vi "01 Dryer_Performance_SM.vi"() -> ()   [LabVIEW 2012] (continued)
        n146 = Concatenate Strings(w279, w280, w267, w263) -> (w272:string)
        n147 = Build Array (concatenate)(w278, w281, w262) -> (w260:string[])
        n148 = String Length(string=w272) -> (length=w277:i32)
        n149 = Decrement(x=w277) -> (x-1=w271:i32)
        n150 = String Subset(string=w272, offset (0)=w271, length (rest)=1 ("length (rest)")) -> (substring=w275:string)
        n151 = Equal?(x=w275, y=",") -> (x = y?=w273:bool)
        n152 = case shown="True" w273 {
          tunnel: w272 -> [w321 w325]
          tunnel: w271 -> [_ w323]
          tunnel: [w321 w322] -> w261
          frame False {
          }
          frame True {
            n153 = String Subset(string=w325, offset (0)=0, length (rest)=w323) -> (substring=w322:string)
          }
        }
        n154 = call "Agilent Sort Channels.vi"("Agilent Chanel List"=w261, "Agilent Label List"=w260) -> ("Sorted Channels"=w259:string, "Sorted Labels Array"=w256:string[])  [unwired: 12 in]
        n155 = local write "DAQ Chanel List"(w259) -> ()
        n156 = Bundle By Name(cluster=w283, "DAQ Chan List"=w259, "DAQ Label List"=w256) -> (w282:T22)
        n157 = call <vilib>:"Add State(s) to Queue__jki_lib_state_machine.vi"("State(s) in (\"\")"=w286) -> ("States Out"=w285:string)  [unwired: 14 in]
        n158 = local write "DAQ Label List"(w256) -> ()
      }
      frame "Initialize CDAQ Channels" {
        # "if ends in , remove it"
        n159 = global read "Global Test Variables DPT.vi" "Globals for Dryer Performance Test"() -> (w336:T9)
        n160 = local read "cDAQ"() -> (w327:bool)
        n161 = Unbundle By Name(w336) -> ("cDAQ Array Locations.Scale Channel"=w335:string, "cDAQ Array Locations.RH Chan"=w334:string, "cDAQ Array Locations.Temp Chan"=w333:string, "Test Setup.Gas Enabled"=w328:bool, "cDAQ Array Locations.Gas Pressure"=w332:string, "cDAQ Array Locations.Gas Temperature"=w331:string, "cDAQ Array Locations.Barometric Pressure"=w330:string, "cDAQ Array Locations.Gas Feedback Chan"=w329:string)
        n162 = call "Panel DPT Channel Test Labels.vi"("CDAQ?"=w327) -> ("Chanel List"=w340:string, "Label Array"=w358:string[])  [unwired: 12 in, 1 out]
        n163 = local write "TC Chanel List"(w340) -> ()
        n164 = local read "USB Weight?"() -> (w345:bool)
        n165 = Search and Replace String(replace all?=TRUE ("replace all? (F)"), input string=w340, search string=",") -> (number of replacements=w347:i32)  [unwired: 5 in, 3 out]
        n166 = call "Panel DPT Voltage Labels.vi"("Chanel List In"=w340, "CDAQ?"=w327, "Label List In"=w358) -> ("Chanel List Out"=w359:string, "Label List Out"=w357:string[], "Stream DC to File(out)?"=→"Stream DC to File?":bool)  [unwired: 10 in]
        n167 = Increment(x=w347) -> (x+1=w339:i32)
        n168 = case shown="False" w345 {
          tunnel: [string[] ["Weight", "Chamber RH", "Chamber Temp"] ("Label List 2") string[] ["cDAQ Weight", "Chamber RH", "Chamber Temp"] ("Label List 2")] -> w365
          tunnel: [w384 w389] -> w346
          tunnel: w335 -> [w382 w388]
          tunnel: w334 -> [w381 w387]
          tunnel: w333 -> [w380 w386]
          frame False {
            w383 = "," ("string")
            n169 = Concatenate Strings(w382, w383, w381, w383, w380) -> (w384:string)
          }
          frame True {
            w390 = "," ("string")
            n170 = Concatenate Strings(w388, w390, w387, w390, w386) -> (w389:string)
          }
        }
        n171 = local write "Number of TCs"(w339) -> ()
        n172 = String Length(string=w359) -> (length=w364:i32)
        n173 = Greater Than 0?(x=w364) -> (x > 0?=w361:bool)
        n174 = Select(t=",", s=w361, f="") -> (s? t:f=w360:string)
        n175 = case shown="True" w328 {
          tunnel: ["" w379] -> w344
          tunnel: [string[] [] ("Label List 2") string[] ["Gas Pressure", "Gas Temperature", "Barometric Pressure", "Gas Feedback"] ("Label List 2")] -> w343
          tunnel: w332 -> [_ w376]
          tunnel: w331 -> [_ w375]
          tunnel: w330 -> [_ w374]
          tunnel: w329 -> [_ w373]
          frame False {
          }
          frame True {
            w377 = "," ("string")
            n176 = Concatenate Strings(w377, w376, w377, w375, w377, w374, w377, w373) -> (w379:string)
          }
        }
        n177 = Concatenate Strings(w359, w360, w346, w344) -> (w351:string)
        n178 = Build Array (concatenate)(w357, w365, w343) -> (w341:string[])
        n179 = String Length(string=w351) -> (length=w356:i32)
        n180 = Decrement(x=w356) -> (x-1=w350:i32)
        n181 = String Subset(string=w351, offset (0)=w350, length (rest)=1 ("length (rest)")) -> (substring=w354:string)
        n182 = Equal?(x=w354, y=",") -> (x = y?=w352:bool)
        n183 = case shown="True" w352 {
          tunnel: w351 -> [w392 w396]
          tunnel: w350 -> [_ w394]
          tunnel: [w392 w393] -> w342
          frame False {
          }
          frame True {
            n184 = String Subset(string=w396, offset (0)=0, length (rest)=w394) -> (substring=w393:string)
          }
        }
        n185 = call "Agilent Sort Channels.vi"("Agilent Chanel List"=w342, "Agilent Label List"=w341) -> ("Sorted Channels"=w338:string, "Sorted Labels Array"=w337:string[])  [unwired: 12 in]
        n186 = Bundle By Name(cluster=w367, "DAQ Chan List"=w338, "DAQ Label List"=w337) -> (w366:T22)
        n187 = call <vilib>:"Add State(s) to Queue__jki_lib_state_machine.vi"("State(s) in (\"\")"=w370) -> ("States Out"=w369:string)  [unwired: 14 in]
        n188 = local write "DAQ Chanel List"(w338) -> ()
        n189 = local write "DAQ Label List"(w337) -> ()
      }
      frame "----Iniialize Equip-----" {
        # "Do not put any code in this frame.\n(It is a separator no-op. You can make a copy of this frame to create a new Data frame)"
        n190 = call <vilib>:"Add State(s) to Queue__jki_lib_state_machine.vi"("State(s) in (\"\")"=w400) -> ("States Out"=w399:string)  [unwired: 14 in]
      }
      frame "Initialize Equipment" {
        w405 = 4  # Invalid IP Address Length Size
        # "Panel to enter drum volume, MA filter, and scale temp coeff.  \nDrum volume needs to be experimentally determined, depending on a heated run with no clothes.\nThis data is processed with anther program.\n(FIXME, maybe automatically generate this?)"
        n191 = global read "Global Test Variables DPT.vi" "Globals for Dryer Performance Test"() -> (w417:T9)
        n192 = Unbundle By Name(w417) -> ("Test Setup.CompVolume"=w402:dbl, "Test Setup.CDAQ"=w413:bool, "Test Setup.34970"=w412:bool, "Test Setup.34980"=w411:bool, "Test Setup.MA Filter Size"=w408:i32, "Test Setup.RH-IP"=w407:string)
        n193 = Unbundle By Name(w428) -> ("Equipment"=w429:T6)
        n194 = String Length(string=w407) -> (length=w406:i32)
        n195 = Greater?(x=w406, y=w405) -> (0:→"ITHX RH Sensor":bool)
        n196 = local read "Use Smoothing"() -> (w418:bool)
        n197 = local write "MA Filter Size"(w408) -> ()
        n198 = Build Array(w413, w412, w411) -> (w410:bool[])
        n199 = Boolean Array To Number(Boolean array=w410) -> (number=w409:u32)
        n200 = case shown="1" w409 {
          tunnel: [" Init: Power Analyzer\nInit: Power\nInit: Gas\nInit: 34970" ("State(s) in Front (\"\")") " Init: Power Analyzer\nInit: Power\nInit: Gas\nInit: CDAQ" ("State(s) in Front (\"\")") " Init: Power Analyzer\nInit: Power\nInit: Gas\nInit: Agilent" ("State(s) in Front (\"\")")] -> w416
          tunnel: [refnum<visa-resource-name> "AGILENT-34970A" ("VISA resource name") refnum<visa-resource-name> "AGILENT-34970" ("VISA resource name") refnum<visa-resource-name> "AGILENT-34980A" ("VISA resource name")] -> w415
          tunnel: [refnum<visa-resource-name> "WT230" ("Com Power") refnum<visa-resource-name> "WT500" ("Com Power") refnum<visa-resource-name> "WT500" ("Com Power")] -> w414
          frame 2, Default {
          }
          frame 1 {
          }
          frame 4 {
          }
        }
        n201 = Bundle By Name(cluster=w429, "Com Agilent"=w415, "Com Flow Computer"=refnum<visa-resource-name> "COM1", "Com Power Meter"=w414, "Com Power Supply"=refnum<visa-resource-name> "CHROMA") -> (w426:T6)
        "Equipment" <- w426
        n202 = disable-structure shown="Enabled" {
          disable-tunnel: w423 -> [w438 _]
          disable-tunnel: [w437 _] -> w422
          disable-tunnel: [w436 0.0 ("Scale Temp Coeff")] -> w421
          disable-tunnel: [w435 13.0 ("Drum Volume")] -> w401
          disable-tunnel: [w434 w439] -> w419
          disable-tunnel: string[][] [["MA Filter Size", "40"], ["Scale Temp Coeff", "0"], ["Drum Volume", "13"]] ("appended array") -> [_ w439]
          disable-tunnel: w402 -> [w433 _]
          frame Enabled {
            n203 = call "Panel Averaging Values.vi"("Default volume value"=w433, "Error In"=w438) -> ("Scale Temp Coeff Out"=w436:dbl, "Drum Volume"=w435:dbl, "Out Strings"=w434:string[][], "Error Out"=w437:errorcluster)  [unwired: 9 in, 1 out]
          }
          frame Disabled {
          }
        }
        n204 = case shown="True" w418 {
          tunnel: [w451 w455] -> w420
          tunnel: w419 -> [w451 w454]
          frame False {
          }
          frame True {
            n205 = Insert Into Array(array=w454, index (row)=0, new element=string[] ["Smoothing Used"] ("new element/subarray")) -> (w455:string[][])  [unwired: 1 in]
          }
        }
        n206 = Bundle By Name(cluster=w428, "Equipment"=w426, "Start Header Data"=w420) -> (w427:T22)
        n207 = local write "Scale Temp Coeff"(w421) -> ()
        n208 = local write "Drum Volume"(w401) -> ()
        n209 = case shown="No Error" w422 {
          selector: w422 -> [_ w457]
          tunnel: [w456 "Macro: Exit" ("State(s) in Front (\"\")")] -> w430
          tunnel: w416 -> [w456 _]
          frame No Error {
          }
          frame Error {
            n210 = call <vilib>:"Simple Error Handler.vi"("error in (no error)"=w457) -> ()  [unwired: 4 in, 5 out]
          }
        }
        n211 = call <vilib>:"Add State(s) to Queue__jki_lib_state_machine.vi"("State(s) in Front (\"\")"=w430, "State(s) in (\"\")"=w432) -> ("States Out"=w431:string)  [unwired: 13 in]
      }
      frame "Init: Power" {
        # "Sets the Chroma power supply output, and reads the voltages with the WT500 to make sure that the \nPower is in range.\n\nOutputs dryer type to globals.  Tests the voltage settings.  Sets the Supply Voltage output variable."
        n212 = local read "Simulate"() -> (w468:bool)
        n213 = Unbundle By Name(w461) -> ("Equipment.Com Power Meter"=w463:refnum<visa-resource-name>, "Equipment.Com Power Supply"=w470:refnum<visa-resource-name>)
        n214 = global read "Global Test Variables DPT.vi" "Globals for Dryer Performance Test"() -> (w462:T9)
        n215 = case shown="False" w468 {
          tunnel: w470 -> [w495 _]
          tunnel: [w491 w541] -> w466
          tunnel: [w484 "120" ("Supply Voltage:")] -> w469
          tunnel: w467 -> [w494 w541]
          tunnel: w463 -> [w493 _]
          tunnel: w462 -> [w487 _]
          tunnel: [w484 "Electric" ("Chroma Power Setting Out")] -> w459
          frame False {
            n216 = call "Panel Power Setting.vi"() -> ("Dryer Type Out"=w485:string, "Chroma Power Setting Out"=w484:string)  [unwired: 14 in]
            n217 = case shown="\"120\", Default" w484 {
              tunnel: [w506 _ w509 w511] -> w479
              tunnel: [TRUE FALSE TRUE TRUE] -> w478
              frame "120", Default {
                w506 = T19[] [enum."Initialize", enum."Output On 120"] items=["Initialize", "Output On 120", "Output On 240", "Output On 208", "Output Off", "Status", "Send Command", "Track Current"]
              }
              frame "NA" {
                # "Skip Init Power"
              }
              frame "208" {
                w509 = T19[] [enum."Initialize", enum."Output On 208"] items=["Initialize", "Output On 120", "Output On 240", "Output On 208", "Output Off", "Status", "Send Command", "Track Current"]
              }
              frame "240" {
                w511 = T19[] [enum."Initialize", enum."Output On 240"] items=["Initialize", "Output On 120", "Output On 240", "Output On 208", "Output Off", "Status", "Send Command", "Track Current"]
              }
            }
            "Use Chroma" <- w478
            n218 = case shown="True" w478 {
              tunnel: w495 -> [_ w500]
              tunnel: w494 -> [w496 w499]
              tunnel: [w496 w498] -> w483
              tunnel: w479 -> [_ w497]
              frame False {
              }
              frame True {
                n219 = for {
                  tunnel: w500 -> [w504]
                  tunnel: w497 -> [w501] mode=indexing
                  shift-right: [w502] -> w498
                  shift-left: w499 -> [w503]
                  n220 = call "Chroma Driver GPIB-VISA-RW.vi"("VISA resource name"=w504, "Chroma Power Select"=w501, "error in (no error)"=w503) -> ("error out"=w502:errorcluster)  [unwired: 11 in, 1 out]
                }
              }
            }
            n221 = call "Delay mS.vi"("Error In"=w483, "milliseconds to wait"=u32 2000) -> ("Error Out"=w481:errorcluster)  [unwired: 13 in]
            n222 = call "WT500 Read Power.vi"("VISA resource name"=w493, "WT500 CMDS"=WT500_Sequences."GetReadings", "error in (no error)"=w481) -> ("Measurement Values"=w492:dbl[], "error out"=w490:errorcluster)  [unwired: 7 in, 4 out]
            n223 = Bundle By Name(cluster=w487, "Test Information.Dryer Type"=w485) -> (w486:T9)
            n224 = case shown="\"240\"" w484 {
              tunnel: w492 -> [w520 w529 w538 _]
              tunnel: [w514 w523 w532 FALSE] -> w489
              frame "240" {
                n225 = Delete From Array(array=w520, length=2, index=0) -> (deleted portion=w517:dbl[])  [unwired: 1 out]
                n226 = In Range and Coerce(upper limit=121.2, x=w517, lower limit=118.8) -> (In Range?=w513:bool[])  [unwired: 1 out]
                n227 = And Array Elements(Boolean array=w513) -> (logical AND=w512:bool)
                n228 = Not(x=w512) -> (.not. x?=w514:bool)
              }
              frame "208" {
                n229 = Delete From Array(array=w529, length=2, index=0) -> (deleted portion=w526:dbl[])  [unwired: 1 out]
                n230 = In Range and Coerce(upper limit=105.2, x=w526, lower limit=102.8) -> (In Range?=w522:bool[])  [unwired: 1 out]
                n231 = And Array Elements(Boolean array=w522) -> (logical AND=w521:bool)
                n232 = Not(x=w521) -> (.not. x?=w523:bool)
              }
              frame "120", Default {
                n233 = Delete From Array(array=w538, length=1, index=0) -> (deleted portion=w535:dbl[])  [unwired: 1 out]
                n234 = In Range and Coerce(upper limit=121.0, x=w535, lower limit=119.0) -> (In Range?=w531:bool[])  [unwired: 1 out]
                n235 = And Array Elements(Boolean array=w531) -> (logical AND=w530:bool)
                n236 = Not(x=w530) -> (.not. x?=w532:bool)
              }
              frame "NA" {
              }
            }
            n237 = global write "Global Test Variables DPT.vi" "Globals for Dryer Performance Test"(w486) -> ()
            n238 = call "Error Bool Add Message.vi"("Error?"=w489, "Message"="Power Out of Range", "Error In"=w490) -> ("Error Out"=w491:errorcluster)  [unwired: 12 in]
          }
          frame True {
          }
        }
        n239 = Bundle By Name(cluster=w461, "Dryer Type"=w459) -> (w460:T22)
        n240 = case shown="Error" w466 {
          tunnel: ["" ("State(s) in Front (\"\")") "Macro: Exit" ("State(s) in Front (\"\")")] -> w465
          tunnel: w464 -> [_ w475]
          frame No Error {
          }
          frame Error {
            n241 = Concatenate Strings("Error:", w475) -> (w477:string)
            n242 = One Button Dialog(message=w477) -> ()  [unwired: 1 in, 1 out]
          }
        }
        n243 = local write "Supply Voltage:"(w469) -> ()
        n244 = call <vilib>:"Add State(s) to Queue__jki_lib_state_machine.vi"("State(s) in Front (\"\")"=w465, "State(s) in (\"\")"=w472) -> ("States Out"=w471:string)  [unwired: 13 in]
      }
      frame "Init: Gas" {
        # "Initializes the gas data for the header.  Also, triggers the bool indicating\nwether gas is going to be used."
        # "(OPEC) and a majority of the natural gas industry in North America have adopted 60 °F and 14.73 psia \nas their standard reference conditions (instead of 60 °F and 14.696 psia) for expressing natural gas volumes and flow rates"
        n245 = global read "Global Test Variables DPT.vi" "Globals for Dryer Performance Test"() -> (w551:T9)
        n246 = Unbundle By Name(w551) -> ("Test Information.Dryer Type"=w550:string)
        n247 = local read "Simulate"() -> (w546:bool)
        n248 = Unbundle By Name(w554) -> ("Start Header Data"=w545:string[][])
        n249 = Equal?(x="Gas", y=w550) -> (x = y?=w543:bool)
        n250 = Compound Arithmetic op=AND(invert w546, w543) -> (w544:bool)
        n251 = property on="Ave Gas Pressure" class="DigNum (strict)"("Visible"=w543) -> ()  [unwired: 2 in, 2 out]
        n252 = case shown="True" w544 {
          tunnel: [w568 w580] -> w557
          tunnel: w558 -> [w568 w579]
          tunnel: [w566 w574] -> w552
          tunnel: [w567 FALSE ("Use Dry Gas Meter Out?")] -> w548
          tunnel: [w567 TRUE ("Use Dry Gas Meter Out?")] -> w547
          tunnel: w545 -> [w566 w576]
          frame False {
            w567 = FALSE ("Use Dry Gas Meter Out?")
          }
          frame True {
            n253 = call "Panel Init Dry Flow Meter.vi"("Error In"=w579) -> ("Heat Val."=w570:dbl, "BTUF3"=w575:string[][], "Error Out"=w580:errorcluster)  [unwired: 12 in]
            n254 = call "Worksheet DOE Audit.vi"() -> ("DOE Data Out"=w573:T23)  [unwired: 8 in, 2 out]
            n255 = Bundle By Name(cluster=w573, "Gas Heat Val"=w570) -> (w572:T23)
            n256 = local read "2015?"() -> (w569:bool)
            n257 = call "Worksheet DOE Audit.vi"("Add?"=TRUE, "DOE Data"=w572, "2015?"=w569) -> ()  [unwired: 5 in, 3 out]
            n258 = Build Array (concatenate)(w576, w575) -> (w574:string[][])
            "BTUF3" <- w574
          }
        }
        "Use Dry Gas Meter?" <- w547
        "Use SL9200 Gas Readings?" <- w548
        n259 = Bundle By Name(cluster=w554, "Start Header Data"=w552) -> (w553:T22)
        n260 = case shown="Error" w557 {
          tunnel: ["" ("State(s) in Front (\"\")") "Macro: Exit" ("State(s) in Front (\"\")")] -> w556
          tunnel: w555 -> [_ w563]
          frame No Error {
          }
          frame Error {
            n261 = Concatenate Strings("Error:", w563) -> (w565:string)
            n262 = One Button Dialog(message=w565) -> ()  [unwired: 1 in, 1 out]
          }
        }
        n263 = call <vilib>:"Add State(s) to Queue__jki_lib_state_machine.vi"("State(s) in Front (\"\")"=w556, "State(s) in (\"\")"=w560) -> ("States Out"=w559:string)  [unwired: 13 in]
      }
      frame "Init: Power Analyzer" {
        # "Initialize WT500."
        n264 = local read "Simulate"() -> (w585:bool)
        n265 = Unbundle By Name(w587) -> ("Equipment.Com Power Meter"=w586:refnum<visa-resource-name>)
        n266 = case shown="False" w585 {
          tunnel: w586 -> [w601 _]
          tunnel: [w596 w602] -> w583
          tunnel: w584 -> [w597 w602]
          frame False {
            w598 = u16 7 items=["AUTO", "500 mA", "1 A", "2 A", "5 A", "10 A", "20 A", "40 A", "S-AUTO", "50 mV", "100 mV", "200 mV", "500 mV", "1 V", "2 V", "5 V", "10 V", "250 mA", "500 mA", "1 A", "2.5 A", "5 A", "10 A", "20 A", "25 mV", "50 mV", "100 mV", "250 mV", "500 mV", "1 V", "2.5 V", "5 V"] ("I Range (7: 40A)")
            w599 = u16 6 items=["AUTO", "15", "30", "60", "100", "150", "300", "600", "1000", "7.5", "15", "30", "50", "75", "150", "300", "500"] ("V Range (8: 1000V)")
            n267 = call "WT500 Read Power.vi"("VISA resource name"=w601, "WT500 CMDS"=WT500_Sequences."Initialize", "V Range (8: 1000V)"=w599, "I Range (7: 40A)"=w598, "error in (no error)"=w597) -> ("Label"=→"Power Label":string[], "error out"=w596:errorcluster)  [unwired: 5 in, 4 out]
          }
          frame True {
          }
        }
        n268 = case shown="Error" w583 {
          tunnel: ["" ("State(s) in Front (\"\")") "Macro: Exit" ("State(s) in Front (\"\")")] -> w582
          tunnel: w581 -> [_ w592]
          frame No Error {
          }
          frame Error {
            n269 = Concatenate Strings("Error:", w592) -> (w594:string)
            n270 = One Button Dialog(message=w594) -> ()  [unwired: 1 in, 1 out]
          }
        }
        n271 = call <vilib>:"Add State(s) to Queue__jki_lib_state_machine.vi"("State(s) in Front (\"\")"=w582, "State(s) in (\"\")"=w589) -> ("States Out"=w588:string)  [unwired: 13 in]
      }
      frame "Init: Agilent" {
        w605 = "," ("string")
        # "RH=chan 3010, 4-20=0-100\nTemp = chan 3011, 4-20 = 32-158"
        n272 = Unbundle By Name(w620) -> ("Equipment.Com Agilent"=w623:refnum<visa-resource-name>, "DAQ Chan List"=w603:string)
        n273 = global read "Global Test Variables DPT.vi" "Globals for Dryer Performance Test"() -> (w616:T9)
        n274 = Unbundle By Name(w616) -> ("Agilent Setup.Scale Channel"=w614:string, "Agilent Setup.TC Channels"=w611:string, "Agilent Setup.VDC Discrete Channels"=w612:string, "Agilent Setup.RH Chan"=w615:string, "Agilent Setup.Temp Chan"=w613:string, "Test Setup.RH Resistor"=w610:dbl, "Test Setup.Temp Resistor"=w609:dbl, "Agilent Setup.Barometric Pressure"=w608:string, "Agilent Setup.Gas Feedback Chan"=w607:string, "Test Setup.Gas P. Resistor"=w606:dbl, "Agilent Setup.Gas Pressure"=w604:string)
        n275 = Concatenate Strings(w615, w605, w613, w605, w607, w605, w604) -> (w617:string)
        n276 = case shown="False" "Simulate" {
          tunnel: w623 -> [w632 _]
          tunnel: w603 -> [w651 _]
          tunnel: w622 -> [w706 w709]
          tunnel: [w629 w709] -> w621
          tunnel: w612 -> [w696 _]
          tunnel: w614 -> [w695 _]
          tunnel: w617 -> [w679 _]
          tunnel: w615 -> [w678 _]
          tunnel: w613 -> [w677 _]
          tunnel: w611 -> [w643 _]
          tunnel: w610 -> [w676 _]
          tunnel: w609 -> [w675 _]
          tunnel: w608 -> [w670 _]
          tunnel: w606 -> [w660 _]
          tunnel: w604 -> [w659 _]
          frame False {
            w639 = T24."10 V" ("Range (5:Auto)")
            n277 = call "AG34980A Initialize.vi"("VISA resource name"=w632, "error in (no error)"=w706) -> ("VISA session"=w708:refnum<visa-resource-name>, "error out"=w707:errorcluster)  [unwired: 12 in]
            n278 = call "AG34980A Reset.vi"("VISA resource name"=w708, "error in (no error)"=w707) -> ("VISA resource name out"=w650:refnum<visa-resource-name>, "error out"=w673:errorcluster)  [unwired: 12 in]
            n279 = call "AG34980A Configure Scale.vi"("VISA resource name"=w650, "Channel List(empty)"=w670, "Gain (1)"=1.5, "error in (no error)"=w673, "Offset (0)"=20.0) -> ("VISA resource name out"=w649:refnum<visa-resource-name>, "error out"=w631:errorcluster)  [unwired: 9 in]
            n280 = call "AG34980A Configure Thermocouple.vi"("VISA resource name"=w649, "Channel List(empty)"=w643, "Reading Units (0:Celcius)"=enum16{"Celcius", "Fahrenheit", "Kelvin"}."Fahrenheit", "Thermocouple Type (2:J-Type)"=T14."T-Type", "Reference Junction Type (2:Fixed)"=enum16{"Internal", "External", "Fixed"}."Internal", "error in (no error)"=w631, "Ref Junction Temperature (0:Manual)"=enum16{"Manual", "Minimum", "Maximum"}."Minimum") -> ("VISA resource name out"=w700:refnum<visa-resource-name>, "error out"=w703:errorcluster)  [unwired: 7 in]
            n281 = call "AG34980A Configure DC Voltage.vi"("VISA resource name"=w700, "Channel List(empty)"=w696, "error in (no error)"=w703) -> ("VISA resource name out"=w705:refnum<visa-resource-name>, "error out"=w704:errorcluster)  [unwired: 11 in]
            n282 = call "AG34980A Configure DC Voltage.vi"("VISA resource name"=w705, "Channel List(empty)"=w695, "Range (5:Auto)"=w639, "error in (no error)"=w704) -> ("VISA resource name out"=w701:refnum<visa-resource-name>, "error out"=w702:errorcluster)  [unwired: 10 in]
            n283 = call "Scale 4-20 sig.vi"("4 mA value"=0.0, "20 mA value"=50.0, "Drop resistor"=w660) -> ("M"=w664:dbl, "B"=w663:dbl)  [unwired: 11 in]
            n284 = call "Scale 4-20 sig.vi"("4 mA value"=0.0, "20 mA value"=100.0, "Drop resistor"=w676) -> ("M"=w687:dbl, "B"=w686:dbl)  [unwired: 11 in]
            n285 = call "AG34980A Configure Scale.vi"("VISA resource name"=w701, "Channel List(empty)"=w695, "Gain (1)"=15.0, "Units (Empty:Default Units)"="LBS", "error in (no error)"=w702, "Offset (0)"=50.0) -> ("VISA resource name out"=w680:refnum<visa-resource-name>, "error out"=w681:errorcluster)  [unwired: 8 in]
            n286 = call "AG34980A Configure DC Voltage.vi"("VISA resource name"=w680, "Channel List(empty)"=w679, "Range (5:Auto)"=w639, "error in (no error)"=w681) -> ("VISA resource name out"=w667:refnum<visa-resource-name>, "error out"=w666:errorcluster)  [unwired: 10 in]
            n287 = call "AG34980A Configure Scale.vi"("VISA resource name"=w667, "Channel List(empty)"=w659, "Gain (1)"=w664, "Units (Empty:Default Units)"="in", "error in (no error)"=w666, "Offset (0)"=w663) -> ("VISA resource name out"=w668:refnum<visa-resource-name>, "error out"=w669:errorcluster)  [unwired: 8 in]
            n288 = call "AG34980A Configure Scale.vi"("VISA resource name"=w668, "Channel List(empty)"=w678, "Gain (1)"=w687, "Units (Empty:Default Units)"="RH", "error in (no error)"=w669, "Offset (0)"=w686) -> ("VISA resource name out"=w692:refnum<visa-resource-name>, "error out"=w691:errorcluster)  [unwired: 8 in]
            n289 = call "Scale 4-20 sig.vi"("4 mA value"=32.0, "20 mA value"=212.0, "Drop resistor"=w675) -> ("M"=w683:dbl, "B"=w682:dbl)  [unwired: 11 in]
            n290 = call "AG34980A Configure Scale.vi"("VISA resource name"=w692, "Channel List(empty)"=w677, "Gain (1)"=w683, "Units (Empty:Default Units)"="F", "error in (no error)"=w691, "Offset (0)"=w682) -> ("VISA resource name out"=w690:refnum<visa-resource-name>, "error out"=w689:errorcluster)  [unwired: 8 in]
            n291 = call "AG34980A Configure Scan.vi"("VISA resource name"=w690, "Scan List(empty)"=w651, "error in (no error)"=w689, "Ordered Scan (F:Off)"=FALSE) -> ("VISA resource name out"=w633:refnum<visa-resource-name>, "error out"=w630:errorcluster)  [unwired: 10 in]
            n292 = call "AG34980A Configure Integration Time.vi"("NPLC Value(6:1PLC)"="NPLC Value(6:1PLC)", "error in (no error)"=w630, "Function (0:DC Volts)"=T13."Temperature", "VISA resource name"=w633) -> ("error out"=w658:errorcluster, "VISA resource name out"=w656:refnum<visa-resource-name>)  [unwired: 6 in]
            n293 = call "AG34980A Display.vi"("error in (no error)"=w658, "Instrument Display (T:On)"=FALSE, "VISA resource name"=w656) -> ("error out"=w642:errorcluster, "VISA resource name out"=w652:refnum<visa-resource-name>)  [unwired: 5 in, 2 out]
            n294 = call "AG34980A Configure Channel Delay.vi"("VISA resource name"=w652, "Channel List"=w651, "Channel Delay Auto (T:Enabled)"="Channel Delay Auto (T:Enabled)", "Channel Delay (sec)"="Channel Delay (sec)", "error in (no error)"=w642) -> ("VISA resource name out"=w645:refnum<visa-resource-name>, "error out"=w644:errorcluster)  [unwired: 9 in]
            n295 = call "AG34980A Temperature Auto Zero.vi"("VISA resource name"=w645, "Channel List(empty)"=w643, "Autozero (0:ON)"="Autozero (0:ON)", "error in (no error)"=w644) -> ("VISA resource name out"=w646:refnum<visa-resource-name>, "error out"=w647:errorcluster)  [unwired: 10 in]
            n296 = call "AG34980A Thermocouple Check.vi"("VISA resource name"=w646, "Channel List(empty)"=w643, "Enable (F:Disable)"="TC Check Enable (F:Disable)", "error in (no error)"=w647) -> ("error out"=w628:errorcluster)  [unwired: 10 in, 1 out]
            n297 = call "AG34980A Error Query (Multiple).vi"("VISA resource name"=w632, "error in (no error)"=w628) -> ("Error Message"=→"Error Message 3":string, "error out"=w629:errorcluster)  [unwired: 10 in, 2 out]
            "3010 resistor" <- w676
            "3011 resistor" <- w675
            "1020 resistor" <- w660
          }
          frame True {
          }
        }
        n298 = local write "DAQ Chanel List"(w603) -> ()
        n299 = case shown="Error" w621 {
          tunnel: ["" ("State(s) in Front (\"\")") "Macro: Exit" ("State(s) in Front (\"\")")] -> w624
          tunnel: w619 -> [_ w711]
          frame No Error {
          }
          frame Error {
            n300 = Concatenate Strings("Error:", w711) -> (w713:string)
            n301 = One Button Dialog(message=w713) -> ()  [unwired: 1 in, 1 out]
          }
        }
        n302 = call <vilib>:"Add State(s) to Queue__jki_lib_state_machine.vi"("State(s) in Front (\"\")"=w624, "State(s) in (\"\")"=w626) -> ("States Out"=w625:string)  [unwired: 13 in]
      }
      frame "Init: 34970" {
        w719 = "116"  # Bar Press
        w720 = "117"  # Gas Vol
        w721 = "114"  # Gas Pres Channel
        w724 = "," ("string")
        # "RH=chan 3010, 4-20=0-100\nTemp = chan 3011, 4-20 = 32-158"
        n303 = global read "Global Test Variables DPT.vi" "Globals for Dryer Performance Test"() -> (w728:T9)
        n304 = Unbundle By Name(w731) -> ("Equipment.Com Agilent"=w734:refnum<visa-resource-name>, "DAQ Chan List"=w723:string)
        n305 = Unbundle By Name(w728) -> ("Test Setup.RH Resistor"=w727:dbl, "Test Setup.Temp Resistor"=w726:dbl, "Test Setup.Gas P. Resistor"=w725:dbl)
        n306 = local read "Simulate"() -> (w722:bool)
        n307 = global read "Global Test Variables DPT.vi" "34970 Weight Chan"() -> (w716:string)
        n308 = global read "Global Test Variables DPT.vi" "34970 TC Chan List"() -> (w718:string)
        n309 = global read "Global Test Variables DPT.vi" "34970 ChTemp Chan"() -> (w715:string)
        n310 = global read "Global Test Variables DPT.vi" "34970 RH Chan"() -> (w717:string)
        n311 = Concatenate Strings(w717, w724, w715, w724, w720, w724, w721) -> (w729:string)
        n312 = case shown="False" w722 {
          tunnel: w734 -> [w740 _]
          tunnel: w723 -> [w742 _]
          tunnel: w733 -> [w792 w795]
          tunnel: [w755 w795] -> w732
          tunnel: w716 -> [w789 _]
          tunnel: w729 -> [w776 _]
          tunnel: w717 -> [w775 _]
          tunnel: w715 -> [w774 _]
          tunnel: w718 -> [w745 _]
          tunnel: w727 -> [w773 _]
          tunnel: w726 -> [w772 _]
          tunnel: w719 -> [_ _]
          tunnel: w725 -> [w762 _]
          tunnel: w721 -> [w761 _]
          frame False {
            n313 = call "Initialize.vi"("VISA Resource Name"=w740, "error in (no error)"=w792) -> ("VISA Resource Name Out"=w794:refnum<visa-resource-name>, "error out"=w793:errorcluster)  [unwired: 12 in]
            n314 = call "Reset.vi"("VISA Resource Name"=w794, "error in (no error)"=w793) -> ("VISA Resource Name Out"=w753:refnum<visa-resource-name>, "error out"=w754:errorcluster)  [unwired: 12 in]
            n315 = call "Conf Temperature.vi"("VISA Resource Name"=w753, "Thermocouple Configuration"=T17 {"Thermocouple Type (Last)"=enum."T", "TC Rjunction (2:Int)"=enum."Internal", "Fixed Rjunction Temp (0:Manual)"=enum."Manual", "TC Auto Check? (F:Don't Check)"=FALSE, "Rjunct Temp Value (0)"=0.0}, "Thermistor Type (3:Last)"=T15."Default (Last)", "error in (no error)"=w754, "Channel List(empty)"=w745, "Units (0:Celsius)"=enum16{"Celsius", "Fahrenheit", "Kelvin"}."Fahrenheit") -> ("VISA Resource Name Out"=w750:refnum<visa-resource-name>, "error out"=w749:errorcluster)  [unwired: 7 in, 1 out]
            n316 = call "Conf Voltage.vi"("VISA Resource Name"=w750, "Range (6:Max)"=T16."10 V", "error in (no error)"=w749, "Channel List (empty)"=w789) -> ("VISA Resource Name Out"=w790:refnum<visa-resource-name>, "error out"=w791:errorcluster)  [unwired: 9 in, 1 out]
            n317 = call "Scale 4-20 sig.vi"("4 mA value"=0.0, "20 mA value"=50.0, "Drop resistor"=w762) -> ("M"=w766:dbl, "B"=w765:dbl)  [unwired: 11 in]
            n318 = call "Scale 4-20 sig.vi"("4 mA value"=0.0, "20 mA value"=100.0, "Drop resistor"=w773) -> ("M"=w784:dbl, "B"=w783:dbl)  [unwired: 11 in]
            n319 = call "Conf Scaling.vi"("VISA Resource Name"=w790, "Gain (1)"=15.0, "Offset (0)"=50.0, "Units (empty)"="LBS" ("Units (Empty:Default Units)"), "error in (no error)"=w791, "Channel List (empty)"=w789) -> ("VISA Resource Name Out"=w777:refnum<visa-resource-name>, "error out"=w778:errorcluster)  [unwired: 7 in, 1 out]
            n320 = call "Conf Voltage.vi"("VISA Resource Name"=w777, "Range (6:Max)"=T16."10 V", "error in (no error)"=w778, "Channel List (empty)"=w776) -> ("VISA Resource Name Out"=w769:refnum<visa-resource-name>, "error out"=w768:errorcluster)  [unwired: 9 in, 1 out]
            n321 = call "Conf Scaling.vi"("VISA Resource Name"=w769, "Gain (1)"=w766, "Offset (0)"=w765, "Units (empty)"="in" ("Units (Empty:Default Units)"), "error in (no error)"=w768, "Channel List (empty)"=w761) -> ("VISA Resource Name Out"=w770:refnum<visa-resource-name>, "error out"=w771:errorcluster)  [unwired: 7 in, 1 out]
            n322 = call "Conf Scaling.vi"("VISA Resource Name"=w770, "Gain (1)"=w784, "Offset (0)"=w783, "Units (empty)"="RH" ("Units (Empty:Default Units)"), "error in (no error)"=w771, "Channel List (empty)"=w775) -> ("VISA Resource Name Out"=w787:refnum<visa-resource-name>, "error out"=w786:errorcluster)  [unwired: 7 in, 1 out]
            n323 = call "Scale 4-20 sig.vi"("4 mA value"=32.0, "20 mA value"=212.0, "Drop resistor"=w772) -> ("M"=w780:dbl, "B"=w779:dbl)  [unwired: 11 in]
            n324 = call "Conf Scaling.vi"("VISA Resource Name"=w787, "Gain (1)"=w780, "Offset (0)"=w779, "Units (empty)"="F" ("Units (Empty:Default Units)"), "error in (no error)"=w786, "Channel List (empty)"=w774) -> ("VISA Resource Name Out"=w741:refnum<visa-resource-name>, "error out"=w743:errorcluster)  [unwired: 7 in, 1 out]
            n325 = call "Conf Scan List.vi"("Scan List (empty)"=w742, "error in (no error)"=w743, "VISA Resource Name"=w741) -> ("error out"=w744:errorcluster, "VISA Resource Name Out"=w739:refnum<visa-resource-name>)  [unwired: 6 in, 1 out]
            n326 = call "Error Query (Multiple).vi"("VISA Resource Name"=w739, "error in (no error)"=w744) -> ("Error Message"=w747:string, "error out"=w755:errorcluster)  [unwired: 10 in, 2 out]
            n327 = local write "Error Message 3"(w747) -> ()
          }
          frame True {
          }
        }
        n328 = local write "DAQ Chanel List"(w723) -> ()
        n329 = case shown="Error" w732 {
          tunnel: ["" ("State(s) in Front (\"\")") "Macro: Exit" ("State(s) in Front (\"\")")] -> w735
          tunnel: w730 -> [_ w797]
          frame No Error {
          }
          frame Error {
            n330 = Concatenate Strings("Error:", w797) -> (w799:string)
            n331 = One Button Dialog(message=w799) -> ()  [unwired: 1 in, 1 out]
          }
        }
        n332 = call <vilib>:"Add State(s) to Queue__jki_lib_state_machine.vi"("State(s) in Front (\"\")"=w735, "State(s) in (\"\")"=w737) -> ("States Out"=w736:string)  [unwired: 13 in]
      }
      frame "Init: CDAQ" {
        # "Do not put any code in this frame.\n(It is a separator no-op. You can make a copy of this frame to create a new Data frame)"
        n333 = local read "CDAQ Tasks"() -> (w808:refnum<k21>[])
        n334 = call "03 cDAQ Chan Tester.vi"("Tasks In"=w808, "error in (no error)"=w809, "Mode"=T18."Init CDAQ") -> ("error out"=w807:errorcluster, "Tasks Out"=w804:refnum<k21>[])  [unwired: 6 in, 1 out]
        n335 = call "Delay mS.vi"("Error In"=w807, "milliseconds to wait"=u32 0) -> ("Error Out"=w802:errorcluster)  [unwired: 13 in]
        n336 = call "03 cDAQ Chan Tester.vi"("Tasks In"=w804, "error in (no error)"=w802, "Mode"=T18."Gather DATA") -> ("error out"=w806:errorcluster, "Tasks Out"=→"CDAQ Tasks":refnum<k21>[])  [unwired: 6 in, 1 out]
        n337 = call <vilib>:"Add State(s) to Queue__jki_lib_state_machine.vi"("State(s) in (\"\")"=w813) -> ("States Out"=w812:string)  [unwired: 14 in]
      }
      frame "Init: Nufi" {
        # "Do not put any code in this frame.\n(It is a separator no-op. You can make a copy of this frame to create a new Data frame)"
        n338 = local read "Nufi?"() -> (w814:bool)
        n339 = case shown="True" w814 {
          frame False {
          }
          frame True {
            n340 = stacked-sequence {
              frame #0 {
                # "Send CMD glabal is reset after the cmd is sent"
                n341 = flat-sequence {
                  frame #0 {
                    w819 = T25 1 items=["CMD_Eval_Mode_Entry_CC1", "CMD_Eval_Mode_Entry_CC2", "CMD_Eval_Mode_Continue", "CMD_Send_DIAG_Info", "CMD_Enable_Debug_Log ", "CMD_Disable_Debug_Log ", "CMD_Send_Log_Data", "CMD_Stop"] ("Command Select")
                    n342 = global write "Nufi Global_ReceivedDataCluster.vi" "Command Select"(w819) -> ()
                  }
                  frame #1 {
                    n343 = global write "Nufi Global_ReceivedDataCluster.vi" "Send CMD"(TRUE) -> ()
                  }
                  frame #2 {
                    n344 = while {
                      stop <- w821 continue-if-true
                      n345 = global read "Nufi Global_ReceivedDataCluster.vi" "Send CMD"() -> (w821:bool)
                      n346 = Wait (ms)(milliseconds to wait=u32 500 ("millisecond multiple")) -> ()  [unwired: 1 out]
                    }
                  }
                }
              }
              frame #1 {
                # "Send CMD glabal is reset after the cmd is sent"
                n347 = flat-sequence {
                  frame #0 {
                    w823 = T25 4 items=["CMD_Eval_Mode_Entry_CC1", "CMD_Eval_Mode_Entry_CC2", "CMD_Eval_Mode_Continue", "CMD_Send_DIAG_Info", "CMD_Enable_Debug_Log ", "CMD_Disable_Debug_Log ", "CMD_Send_Log_Data", "CMD_Stop"] ("Command Select")
                    n348 = global write "Nufi Global_ReceivedDataCluster.vi" "Command Select"(w823) -> ()
                  }
                  frame #1 {
                    n349 = global write "Nufi Global_ReceivedDataCluster.vi" "Send CMD"(TRUE) -> ()
                  }
                  frame #2 {
                    n350 = while {
                      stop <- w825 continue-if-true
                      n351 = global read "Nufi Global_ReceivedDataCluster.vi" "Send CMD"() -> (w825:bool)
                      n352 = Wait (ms)(milliseconds to wait=u32 500 ("millisecond multiple")) -> ()  [unwired: 1 out]
                    }
                  }
                }
              }
            }
          }
        }
        n353 = call <vilib>:"Add State(s) to Queue__jki_lib_state_machine.vi"("State(s) in (\"\")"=w818) -> ("States Out"=w817:string)  [unwired: 14 in]
      }
      frame "Init Complete" {
        n354 = flat-sequence {
          frame #0 {
            n355 = Wait (ms)(milliseconds to wait=u32 2000) -> ()  [unwired: 1 out]
          }
          frame #1 {
            w833 = TRUE ("Init Complete")
            n356 = property on="Loggin Data" class="Bool (strict)"("Val(Sgnl)"=w833) -> ()  [unwired: 2 in, 2 out]
            "Loggin Data" <- w833
          }
        }
        n357 = call "String_in_Reference.vi"("String"="Starting Test Log..." ("string")) -> ()  [unwired: 18 in, 1 out]
        n358 = call <vilib>:"Add State(s) to Queue__jki_lib_state_machine.vi"("State(s) in (\"\")"=w831) -> ("States Out"=w830:string)  [unwired: 14 in]
      }
      frame "-----Start Sequence----" {
        # "Do not put any code in this frame.\n(It is a separator no-op. You can make a copy of this frame to create a new Data frame)"
        n359 = call <vilib>:"Add State(s) to Queue__jki_lib_state_machine.vi"("State(s) in (\"\")"=w837) -> ("States Out"=w836:string)  [unwired: 14 in]
      }
      frame "Start: Dryer Info" {
        # "2.2 Ambient temperature and humidity. Maintain the room ambient air temperature at 75 ±3 °F and the room relative humidity at 50\n±10 percent relative humidity"
        # "Before any test cycle, operate the dryer without a test load in the non-heat mode for 15 minutes\nor until the discharge air temperature is varying less than 1 °F for 10 minutes, which ever is longer, in the test installation location\nwith the ambient conditions within the specified rest condition tolerances of 2.2."
        n360 = local read "cDAQ"() -> (w838:bool)
        n361 = local read "Simulate"() -> (w848:bool)
        n362 = global read "Global Test Variables DPT.vi" "Globals for Dryer Performance Test"() -> (w841:T9)
        n363 = Unbundle By Name(w841) -> ("Agilent Setup.RDB Channel"=w842:string)
        n364 = Unbundle By Name(w846) -> ("Equipment.Com Power Supply"=w839:refnum<visa-resource-name>, "Equipment"=w843:T6)  [unwired: 1 out]
        n365 = case shown="False" w848 {
          tunnel: w849 -> [w862 w896]
          tunnel: [w875 100.0 ("Cold Dryer Weight")] -> w840
          tunnel: w843 -> [w864 _]
          tunnel: w842 -> [w874 _]
          tunnel: w839 -> [w869 _]
          tunnel: [w867 w896] -> w847
          tunnel: w838 -> [w866 _]
          frame False {
            n366 = call "Worksheet DOE Audit.vi"() -> ("DOE Data Out"=w860:T23)  [unwired: 8 in, 2 out]
            n367 = local read "CDAQ Tasks"() -> (w863:refnum<k21>[])
            n368 = call "Off Mode Standby Mode Power Measure SM.vi"("Equipment"=w864, "CDAQ Tasks"=w863, "Error In"=w862) -> ("Off Mode Watts"=w856:dbl, "2015 Output"=w857:bool, "Standby Watts"=w855:dbl, "Low Power Switch"=→"Low Power Switch":bool, "Error Out"=w861:errorcluster)  [unwired: 8 in]
            "2015?" <- w857
            n369 = Bundle By Name(cluster=w860, "Off Mode Power"=w856, "Standby Power"=w855) -> (w859:T23)
            n370 = call "Worksheet DOE Audit.vi"("Add?"=TRUE, "DOE Data"=w859, "2015?"=w857) -> ()  [unwired: 5 in, 3 out]
            n371 = call "Dryer PreCondition SM.vi"("Equipment"=w864, "CDAQ Tasks"=w863, "RDB Channel"=w874, "CDAQ?"=w866, "Error In"=w861) -> ("Cold Dryer Weight"=w875:dbl, "Error Out"=w868:errorcluster)  [unwired: 9 in]
            n372 = local read "Supply Voltage:"() -> (w873:string)
            n373 = case shown="\"120\", Default" w873 {
              tunnel: [Chroma_Driver_Select."Output On 120" ("Chroma Power Select") Chroma_Driver_Select."Output On 208" ("Chroma Power Select") Chroma_Driver_Select."Output On 240" ("Chroma Power Select")] -> w871
              frame "120", Default {
              }
              frame "208 " {
              }
              frame "240" {
              }
            }
            n374 = local read "Use Chroma"() -> (w865:bool)
            n375 = Build Array(Chroma_Driver_Select."Output Off" ("Chroma Power Select"), w871) -> (w870:T19[])
            n376 = case shown="True" w865 {
              tunnel: w870 -> [_ w880]
              tunnel: w869 -> [_ w879]
              tunnel: w868 -> [w876 w878]
              tunnel: [w876 w877] -> w867
              frame False {
              }
              frame True {
                n377 = for {
                  tunnel: w879 -> [w887]
                  tunnel: w880 -> [w884] mode=indexing
                  shift-right: [w883] -> w877
                  shift-left: w878 -> [w886]
                  i -> [w882]
                  n378 = call "Chroma Driver GPIB-VISA-RW.vi"("VISA resource name"=w887, "Chroma Power Select"=w884, "error in (no error)"=w886) -> ("error out"=w885:errorcluster)  [unwired: 11 in, 1 out]
                  n379 = Equal To 0?(x=w882) -> (x = 0?=w881:bool)
                  n380 = case shown="False" w881 {
                    tunnel: w885 -> [w888 w891]
                    tunnel: [w888 w890] -> w883
                    frame False {
                    }
                    frame True {
                      n381 = call "Delay mS.vi"("Error In"=w891, "milliseconds to wait"=u32 7000) -> ("Error Out"=w890:errorcluster)  [unwired: 13 in]
                    }
                  }
                }
              }
            }
          }
          frame True {
          }
        }
        "Empty Dryer Cold Weight" <- w840
        n382 = Bundle By Name(cluster=w841, "Test Information.Empty Dryer Cold Weight:"=w840) -> (w844:T9)
        n383 = Bundle By Name(cluster=w846, "Empty Dryer Cold Weight"=w840) -> (w845:T22)
        n384 = global write "Global Test Variables DPT.vi" "Globals for Dryer Performance Test"(w844) -> ()
        n385 = case shown="Error" w847 {
          tunnel: ["" ("State(s) in Front (\"\")") "Macro: Exit" ("State(s) in Front (\"\")")] -> w851
          tunnel: w850 -> [_ w899]
          frame No Error {
          }
          frame Error {
            n386 = Concatenate Strings("Error:", w899) -> (w901:string)
            n387 = One Button Dialog(message=w901) -> ()  [unwired: 1 in, 1 out]
          }
        }
        n388 = call <vilib>:"Add State(s) to Queue__jki_lib_state_machine.vi"("State(s) in Front (\"\")"=w851, "State(s) in (\"\")"=w853) -> ("States Out"=w852:string)  [unwired: 13 in]
      }
      frame "Start: Gas Reading" {
        n389 = local read "Simulate"() -> (w910:bool)
        n390 = global read "Global Test Variables DPT.vi" "Globals for Dryer Performance Test"() -> (w905:T9)
        n391 = Unbundle By Name(w905) -> ("Test Information.Dryer Type"=w906:string)
        n392 = Not Equal?(x="Gas", y=w906) -> (x != y?=w902:bool)
        n393 = Or(x=w902, y=w910) -> (x .or. y?=w903:bool)
        n394 = case shown="False" w903 {
          tunnel: w911 -> [w917 w966]
          tunnel: [w917 w966] -> w907
          tunnel: w909 -> [w929 _]
          tunnel: w909 -> [w924 w965]
          tunnel: [w923 w965] -> w908
          frame False {
            n395 = local read "cDAQ"() -> (w916:bool)
            n396 = Unbundle By Name(w929) -> ("Start Header Data"=w922:string[][], "Equipment.Com Agilent"=w918:refnum<visa-resource-name>)
            n397 = case shown="False" w916 {
              tunnel: [w945 w962] -> w928
              tunnel: [w944 w961] -> w927
              tunnel: w918 -> [_ w955]
              frame True {
                n398 = global read "Global Test Variables DPT.vi" "Globals for Dryer Performance Test"() -> (w936:T9)
                n399 = Unbundle By Name(w936) -> ("cDAQ Array Locations.Gas Feedback Chan"=w935:string)
                n400 = local read "CDAQ Tasks"() -> (w932:refnum<k21>[])
                n401 = call "Panel Reset Gas Vol.vi"("Tasks In"=w932) -> ("CDAQ Data Out"=w931:dbl[])  [unwired: 10 in]
                "CDAQ Data Out" <- w931
                n402 = Decimal String To Number(string=w935) -> (number=w934:i32)  [unwired: 2 in, 1 out]
                n403 = Index Array(array=w931, index=w934) -> (element=w933:dbl)
                n404 = Number To Fractional String(number=w933, precision (6)=i16 3) -> (F-format string=w938:string)  [unwired: 2 in]
                n405 = Fract/Exp String To Number(string=w938) -> (number=w939:dbl)  [unwired: 3 in, 1 out]
                n406 = local read "2015?"() -> (w930:bool)
                n407 = call "Worksheet DOE Audit.vi"() -> ("DOE Data Out"=w942:T23)  [unwired: 8 in, 2 out]
                n408 = Bundle By Name(cluster=w942, "Gas Vol Init"=w939) -> (w941:T23)
                n409 = Build Array(w938) -> (w945:string[])
                n410 = Build Array("Dry Meter Initial Reading") -> (w944:string[])
                n411 = call "Worksheet DOE Audit.vi"("Add?"=TRUE, "DOE Data"=w941, "2015?"=w930) -> ()  [unwired: 5 in, 3 out]
              }
              frame False {
                n412 = global read "Global Test Variables DPT.vi" "Globals for Dryer Performance Test"() -> (w954:T9)
                n413 = flat-sequence {
                  tunnel: [T20."10 V" ("Range (5:Auto)")] -> w947
                  frame #0 {
                    n414 = One Button Dialog(message="Reset Gas Volume") -> ()  [unwired: 1 in, 1 out]
                  }
                }
                n415 = Unbundle By Name(w954) -> ("Agilent Setup.Gas Feedback Chan"=w953:string)
                n416 = call "AG34980A Measure DC Voltage.vi"("VISA resource name"=w955, "Channel List(empty)"=w953, "Range (5:Auto)"=w947) -> ("Output Array"=w952:dbl[])  [unwired: 10 in, 2 out]
                n417 = Array To Cluster(array=w952) -> (cluster=w951:cluster{"Output Array[0]":dbl})
                n418 = Unbundle(w951) -> ("Output Array[0]"=w949:dbl)
                n419 = Number To Fractional String(number=w949, precision (6)=i16 3) -> (F-format string=w950:string)  [unwired: 2 in]
                n420 = Fract/Exp String To Number(string=w950) -> (number=w956:dbl)  [unwired: 3 in, 1 out]
                n421 = local read "2015?"() -> (w946:bool)
                n422 = call "Worksheet DOE Audit.vi"() -> ("DOE Data Out"=w959:T23)  [unwired: 8 in, 2 out]
                n423 = Bundle By Name(cluster=w959, "Gas Vol Init"=w956) -> (w958:T23)
                n424 = Build Array("Dry Meter Initial Reading") -> (w961:string[])
                n425 = Build Array(w950) -> (w962:string[])
                n426 = call "Worksheet DOE Audit.vi"("Add?"=TRUE, "DOE Data"=w958, "2015?"=w946) -> ()  [unwired: 5 in, 3 out]
              }
            }
            n427 = Build Array (concatenate)(w928) -> (w925:string[])
            n428 = Build Array (concatenate)(w927) -> (w926:string[])
            n429 = Build Array(w926, w925) -> (w920:string[][])
            n430 = Transpose 2D Array(2D array=w920) -> (transposed array=w919:string[][])
            n431 = Build Array (concatenate)(w922, w919) -> (w921:string[][])
            n432 = Bundle By Name(cluster=w924, "Start Header Data"=w921) -> (w923:T22)
          }
          frame True {
          }
        }
        n433 = case shown="Error" w907 {
          tunnel: ["" ("State(s) in Front (\"\")") "Macro: Exit" ("State(s) in Front (\"\")")] -> w913
          tunnel: w912 -> [_ w969]
          frame No Error {
          }
          frame Error {
            n434 = Concatenate Strings("Error:", w969) -> (w971:string)
            n435 = One Button Dialog(message=w971) -> ()  [unwired: 1 in, 1 out]
          }
        }
        n436 = call <vilib>:"Add State(s) to Queue__jki_lib_state_machine.vi"("State(s) in Front (\"\")"=w913, "State(s) in (\"\")"=w915) -> ("States Out"=w914:string)  [unwired: 13 in]
      }
      frame "Start: Ambient" {
        n437 = local read "Simulate"() -> (w975:bool)
        n438 = case shown="False" w975 {
          tunnel: w976 -> [w999 w1057]
          tunnel: [w998 w1057] -> w972
          tunnel: w974 -> [w1009 _]
          tunnel: w974 -> [w1008 w1056]
          tunnel: [w1007 w1056] -> w973
          frame False {
            n439 = local read "ITHX RH Sensor"() -> (w982:bool)
            n440 = global read "Global Test Variables DPT.vi" "Globals for Dryer Performance Test"() -> (w1001:T9)
            n441 = Unbundle By Name(w1009) -> ("Start Header Data"=w1006:string[][], "Equipment.Com Agilent"=w1000:refnum<visa-resource-name>, "DAQ Label List"=w994:string[])  [unwired: 1 out]
            n442 = Unbundle By Name(w1001) -> ("cDAQ Array Locations.RH Chan"=w984:string, "cDAQ Array Locations.Temp Chan"=w983:string)
            n443 = case shown="False" w982 {
              tunnel: w1000 -> [w1018 _]
              tunnel: w999 -> [w1017 w1055]
              tunnel: [w1016 w1054] -> w998
              tunnel: w994 -> [w1015 _]
              tunnel: [w1014 w1048] -> w989
              tunnel: [w1013 w1049] -> w986
              tunnel: w984 -> [w1012 _]
              tunnel: w983 -> [w1011 _]
              frame False {
                n444 = local read "cDAQ"() -> (w1010:bool)
                n445 = case shown="True" w1010 {
                  tunnel: w1018 -> [w1036 _]
                  tunnel: w1017 -> [w1035 w1039]
                  tunnel: [w1022 w1038] -> w1016